vi "VNA-FMR-POLREF_(LV2017).vi"() -> ()   [LabVIEW 2017] (continued)
  out "XY Graph 3":cluster{"Trace Data":dbl[], "Trace Data":dbl[]}(graph)
  in  "RF State (T) 2":bool=TRUE caption="RF State (T)"
  in  "Bandwidth":dbl=400.0 caption="Bandwidth (10.0e3)" format="%#.9p"
  in  "Sweep Time":dbl=8.0 caption="Sweep Time (21.909e-3)" format="%^.3e"
  in  "Auto Sweep Time":bool caption="Auto Sweep Time (T)"
  in  "Power":dbl=-2.0 caption="Power (-10.0)" format="%^.3e"
  in  "Number Of Points":i32=1601
  in  "Display 2":bool=TRUE
  out "Current value":dbl=0.2540000081062317
  out "Range 4":dbl
  out "Units 6":dbl
  out "Mode 4":dbl=1.0
  in  "Commit 2":bool caption="Commit"
  out "Formatted value":dbl=0.2540000081062317 format="%3_4p"
  out "Units 5":string="T"
  in  "Range 3":i32(knob) scale=0.0..4.0
  in  "Mode 3":u32(knob) scale=0.0..4.0
  in  "Units 4":u32(knob) scale=0.0..3.0
  out "Ba Stability":string="wait"
  out "Actual Current Level (A)":dbl=8.81 format="%.2g"
  out "output matrix 2":T1
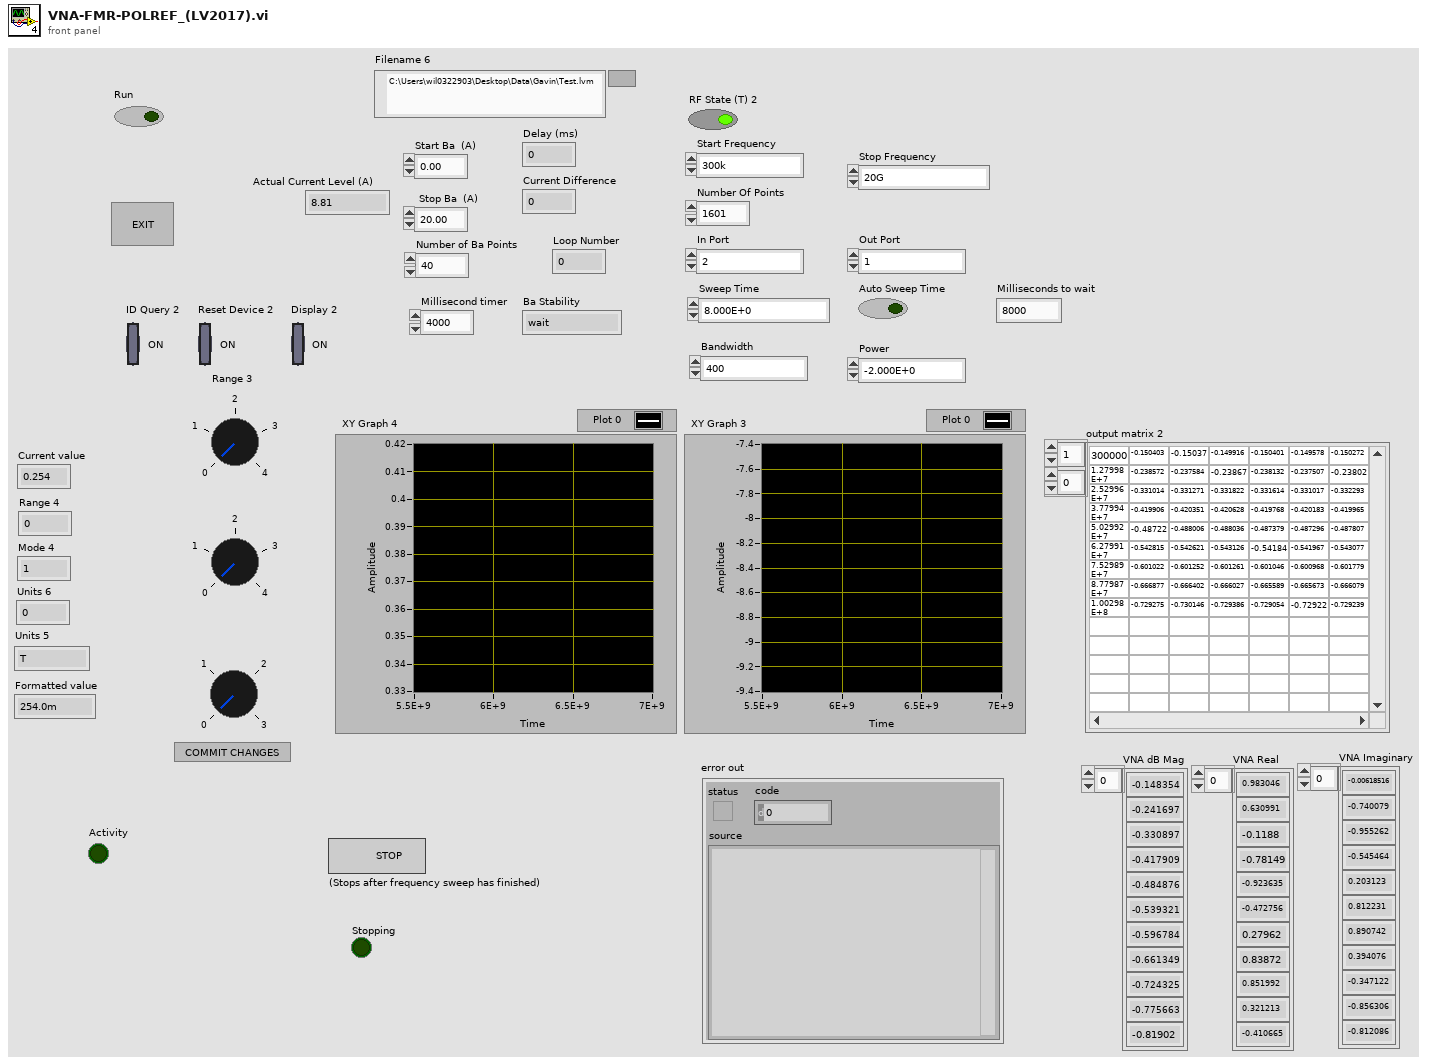
[diagram p1: front panel]
types:
  T1 = typedef "NI_Matrix.lvlib/RealMatrix.ctl" = dbl[][]
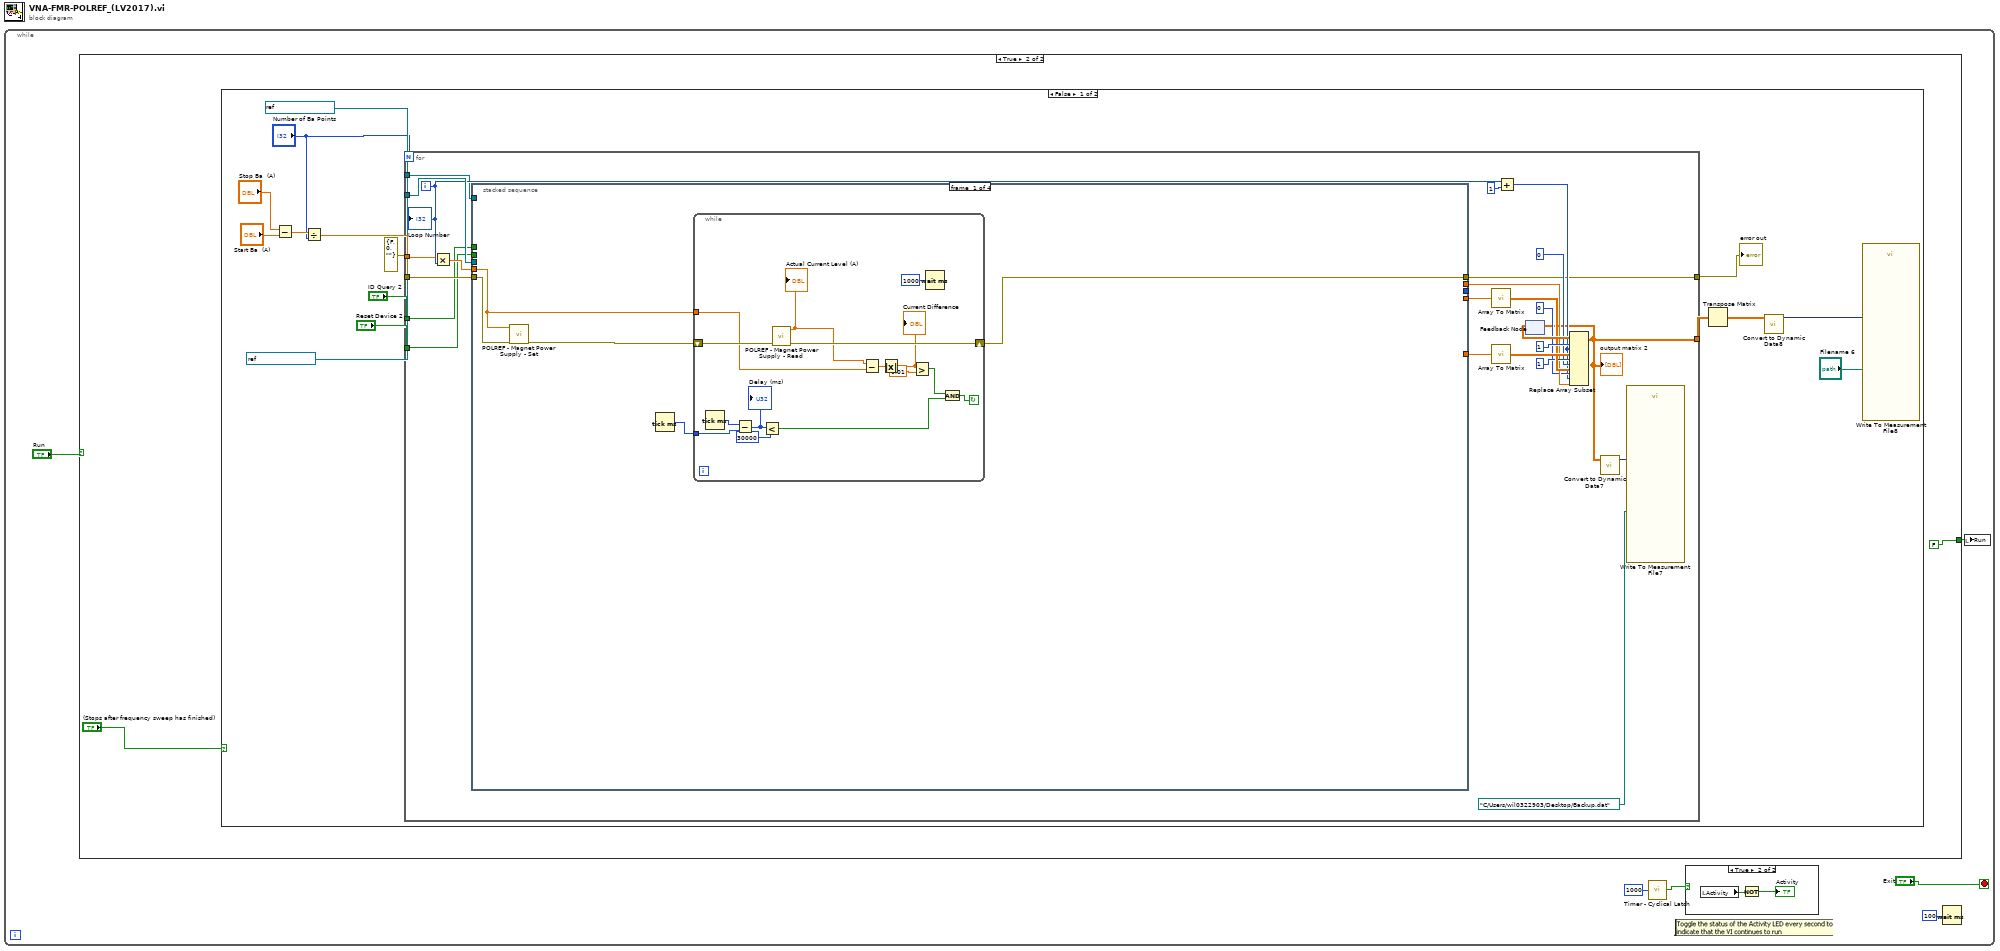
[diagram p0: block diagram]
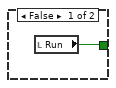
[diagram p3: hidden frame]
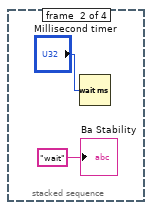
[diagram p4: hidden frame]
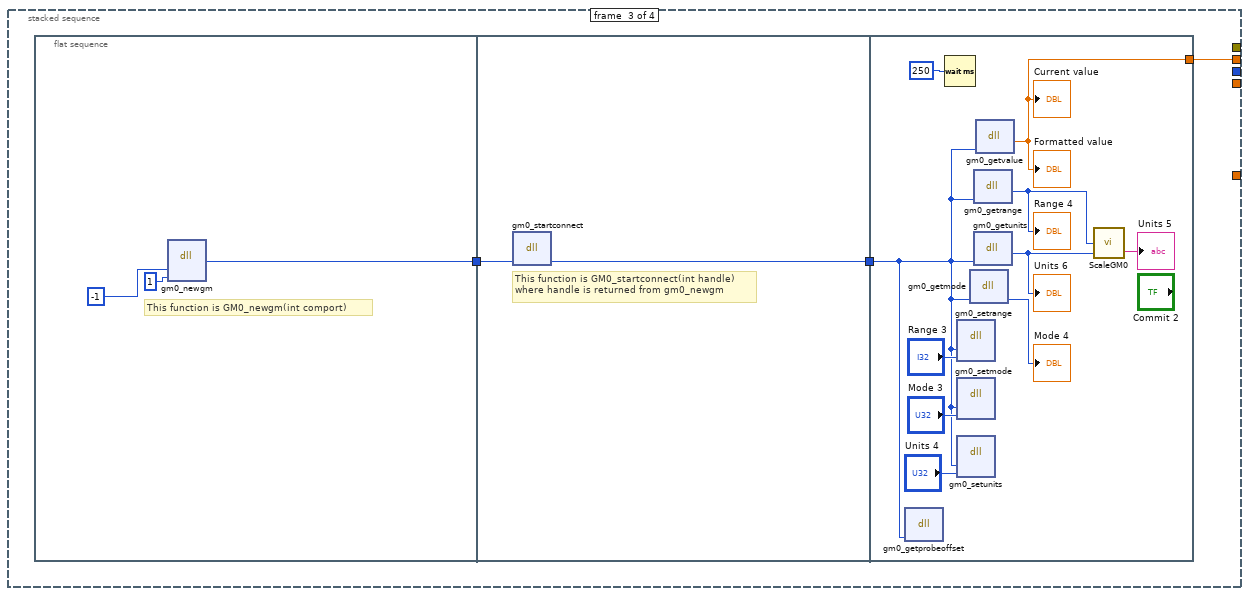
[diagram p5: hidden frame]
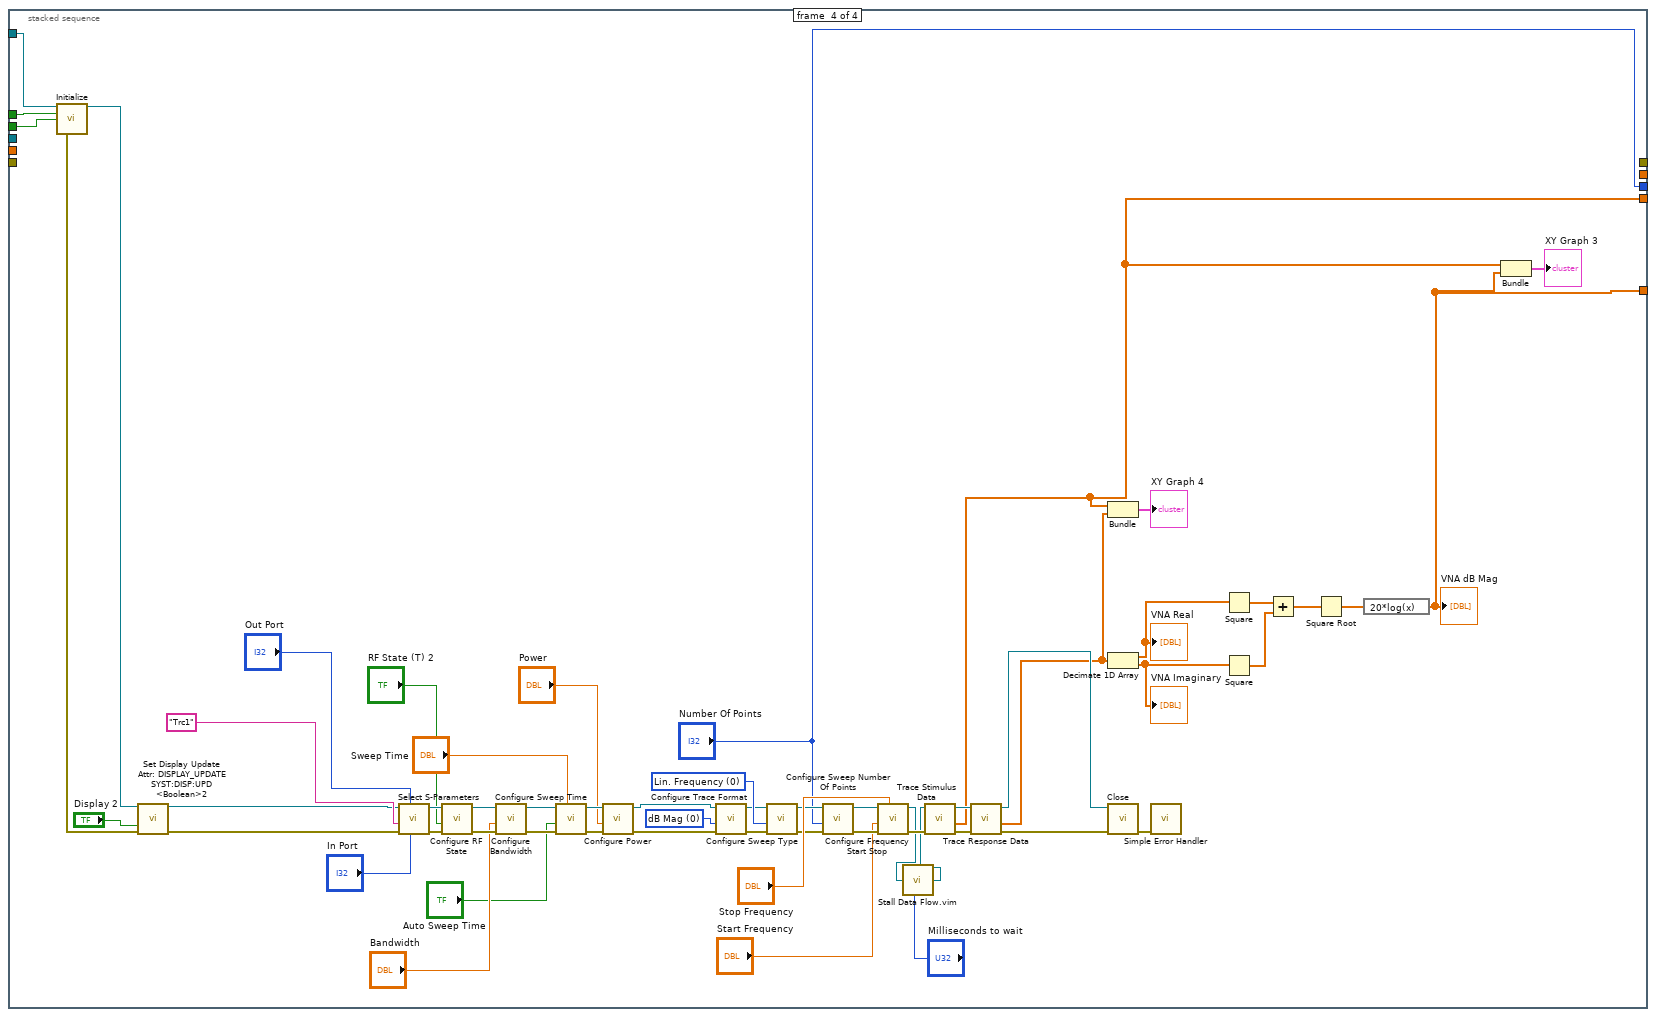
[diagram p6: hidden frame]
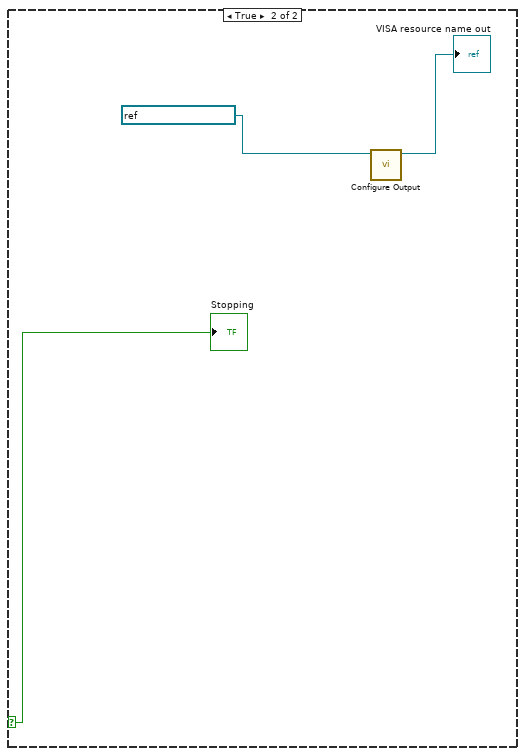
[diagram p7: hidden frame]
diagram:
  n1 = while {
    stop <- "Exit" stop-if-true
    n2 = case shown="True" "Run" {
      tunnel: [w9 FALSE ("Run Button")] -> w1
      frame False {
        n3 = local read "Run"() -> (w9:bool)
      }
      frame True {
        n4 = case shown="False" "(Stops after frequency sweep has finished)" {
          selector: "(Stops after frequency sweep has finished)" -> [_ w150]
          frame False {
            n5 = Subtract(x="Stop Ba  (A)", y="Start Ba  (A)") -> (x-y=w18:dbl)
            n6 = Divide(x=w18, y="Number of Ba Points") -> (x/y=w16:dbl)
            n7 = for {
              N: "Number of Ba Points" -> [_]
              tunnel: [w36] -> w24
              tunnel: w16 -> [w32]
              tunnel: errorcluster {"status"=FALSE, "code"=0, "source"=""} ("error in (no error)") -> [w35]
              tunnel: refnum<visa-resource-name> "GPIB1::11::INSTR" ("VISA resource name 3") -> [w34]
              tunnel: refnum<visa-resource-name> "GPIB1::20::INSTR" ("VISA resource name 2") -> [w30]
              tunnel: "ID Query 2" -> [w29]
              tunnel: "Reset Device 2" -> [w28]
              tunnel: [w27] -> w12
              i -> [w33]
              n8 = Multiply(x=w32, y=w33) -> (x*y=w31:dbl)
              n9 = stacked-sequence {
                tunnel: [_ _ w73 _] -> w41
                tunnel: [_ _ _ w104] -> w49
                tunnel: [_ _ _ w103] -> w50
                tunnel: [_ _ _ "Number Of Points"] -> _
                tunnel: w34 -> [_ _ _ _]
                tunnel: w35 -> [w55 _ _ _]
                tunnel: w31 -> [w52 _ _ _]
                tunnel: w30 -> [_ _ _ w99]
                tunnel: w29 -> [_ _ _ w98]
                tunnel: w28 -> [_ _ _ w97]
                tunnel: [w53 _ _ _] -> w27
                frame #0 {
                  n10 = call "POLREF - Magnet Power Supply - Set.vi"("error in (no error)"=w55, "Magnet Current - Set"=w52) -> ("error out"=w54:errorcluster)  [unwired: 9 in]
                  n11 = Tick Count (ms)() -> (millisecond timer value=w51:u32)
                  n12 = while {
                    shift-right: [w69] -> w53
                    shift-left: w54 -> [w70]
                    tunnel: w52 -> [w67]
                    tunnel: w51 -> [w61]
                    stop <- w57 continue-if-true
                    n13 = Tick Count (ms)() -> (millisecond timer value=w62:u32)
                    n14 = Subtract(x=w62, y=w61) -> (x-y=w60:u32)
                    "Delay (ms)" <- w60
                    n15 = Less?(x=w60, y=u32 30000) -> (x < y?=w58:bool)
                    n16 = call "POLREF - Magnet Power Supply - Read.vi"("error in (no error)"=w70) -> ("error out"=w69:errorcluster, "Magnet Current"=w68:dbl)  [unwired: 9 in]
                    "Actual Current Level (A)" <- w68
                    n17 = Subtract(x=w68, y=w67) -> (x-y=w66:dbl)
                    n18 = Absolute Value(x=w66) -> (abs(x)=w65:dbl)
                    "Current Difference" <- w65
                    n19 = Greater?(x=w65, y=0.01) -> (0:w56:bool)
                    n20 = Wait (ms)(milliseconds to wait=u32 1000) -> ()  [unwired: 1 out]
                    n21 = Compound Arithmetic op=AND(w56, w58) -> (w57:bool)
                  }
                }
                frame #1 {
                  n22 = Wait (ms)(milliseconds to wait="Millisecond timer") -> ()  [unwired: 1 out]
                  "Ba Stability" <- "wait"
                }
                frame #2 {
                  n23 = flat-sequence {
                    tunnel: [w76] -> w75
                    tunnel: w75 -> [w79]
                    tunnel: [w80] -> w74
                    tunnel: w74 -> [w82]
                    tunnel: [w81] -> w73
                    frame #0 {
                      # "This function is GM0_newgm(int comport)"
                      n24 = dll-call lib="C:/Users/wil0322903/Desktop/Hall Probe/LabView-VI/gm0.dll" fn="gm0_newgm"("comport"=-1 ("Com Port 2"), "mode"=1) -> ("handle"=w76:i32)  [unwired: 5 in, 2 out]
                    }
                    frame #1 {
                      # "This function is GM0_startconnect(int handle)\nwhere handle is returned from gm0_newgm"
                      n25 = dll-call lib="C:/Users/wil0322903/Desktop/Hall Probe/LabView-VI/gm0.dll" fn="gm0_startconnect"("handle"=w79) -> ("handle"=w80:i32)  [unwired: 4 in, 2 out]
                    }
                    frame #2 {
                      n26 = dll-call lib="C:/Users/wil0322903/Desktop/Hall Probe/LabView-VI/gm0.dll" fn="gm0_getprobeoffset"("handle"=w82) -> ()  [unwired: 5 in, 2 out]
                      n27 = Wait (ms)(milliseconds to wait=250) -> ()  [unwired: 1 out]
                      n28 = dll-call lib="C:/Users/wil0322903/Desktop/Hall Probe/LabView-VI/gm0.dll" fn="gm0_setrange"("handle"=w82, "new range"="Range 3") -> ()  [unwired: 6 in, 2 out]
                      n29 = dll-call lib="C:/Users/wil0322903/Desktop/Hall Probe/LabView-VI/gm0.dll" fn="gm0_setmode"("handle"=w82, "new mode"="Mode 3") -> ()  [unwired: 6 in, 2 out]
                      n30 = dll-call lib="C:/Users/wil0322903/Desktop/Hall Probe/LabView-VI/gm0.dll" fn="gm0_setunits"("handle"=w82, "new units"="Units 4") -> ()  [unwired: 6 in, 2 out]
                      n31 = dll-call lib="C:/Users/wil0322903/Desktop/Hall Probe/LabView-VI/gm0.dll" fn="gm0_getmode"("handle"=w82) -> ("handle"=→"Mode 4":i32)  [unwired: 4 in, 2 out]
                      n32 = dll-call lib="C:/Users/wil0322903/Desktop/Hall Probe/LabView-VI/gm0.dll" fn="gm0_getrange"("handle"=w82) -> ("value"=w88:i32)  [unwired: 4 in, 2 out]
                      "Range 4" <- w88
                      n33 = dll-call lib="C:/Users/wil0322903/Desktop/Hall Probe/LabView-VI/gm0.dll" fn="gm0_getunits"("handle"=w82) -> ("units"=w87:i32)  [unwired: 4 in, 2 out]
                      "Units 6" <- w87
                      n34 = dll-call lib="C:/Users/wil0322903/Desktop/Hall Probe/LabView-VI/gm0.dll" fn="gm0_getvalue"("handle"=w82) -> ("value"=w81:dbl)  [unwired: 4 in, 2 out]
                      "Current value" <- w81
                      "Formatted value" <- w81
                      n35 = call "ScaleGM0.vi"("Units"=w87, "Range"=w88) -> ("Units"=→"Units 5":string)  [unwired: 1 in, 1 out]
                    }
                  }
                }
                frame #3 {
                  w141 = 0 items=["Lin. Frequency", "Log. Frequency", "Segmented Frequency", "Power", "Time", "CW Mode"] ("Sweep Type (Power)")
                  w142 = 0 items=["dB Mag", "Phase", "Smith", "Polar", "Delay", "SWR", "Lin Mag", "Real", "Imag", "Inverted Smith", "Unwrapped Phase"] ("Format (dB Mag)")
                  n36 = call <instrlib>:"Initialize.vi"("VISA resource name"=w99, "ID Query (T: Check)"=w98, "Reset (T: Reset)"=w97) -> ("VISA resource name out"=w94:refnum<visa-resource-name>, "error out"=w101:errorcluster)  [unwired: 11 in]
                  n37 = call "Set Display Update \nAttr: DISPLAY_UPDATE\nSYST:DISP:UPD <Boolean>2"("instrument handle"=w94, "Display Update (OFF)"="Display 2", "error in (no error)"=w101) -> ("instrument handle out"=w96:refnum<visa-resource-name>, "error out"=w95:errorcluster)  [unwired: 11 in]
                  n38 = call <instrlib>:"Select S-Parameters.vi"("In Port (1)"="In Port", "Out Port (1)"="Out Port", "error in (no error)"=w95, "Trace Name (\"Trc1\")"="Trc1" ("Trace Name (\"Trc1\") 2"), "VISA resource name"=w96) -> ("error out"=w116:errorcluster, "VISA resource name out"=w119:refnum<visa-resource-name>)  [unwired: 5 in]
                  n39 = call <instrlib>:"Configure RF State.vi"("error in (no error)"=w116, "RF State (T)"="RF State (T) 2", "VISA resource name"=w119) -> ("error out"=w115:errorcluster, "VISA resource name out"=w118:refnum<visa-resource-name>)  [unwired: 7 in]
                  n40 = call <instrlib>:"Configure Bandwidth.vi"("error in (no error)"=w115, "Bandwidth (10kHz)"="Bandwidth", "VISA resource name"=w118) -> ("error out"=w114:errorcluster, "VISA resource name out"=w117:refnum<visa-resource-name>)  [unwired: 7 in]
                  n41 = call <instrlib>:"Configure Sweep Time.vi"("Sweep Time (21.909e-3)"="Sweep Time", "error in (no error)"=w114, "Auto Sweep Time (T)"="Auto Sweep Time", "VISA resource name"=w117) -> ("error out"=w108:errorcluster, "VISA resource name out"=w109:refnum<visa-resource-name>)  [unwired: 6 in]
                  n42 = call <instrlib>:"Configure Power.vi"("error in (no error)"=w108, "Power (-10.0)"="Power", "VISA resource name"=w109) -> ("error out"=w106:errorcluster, "VISA resource name out"=w107:refnum<visa-resource-name>)  [unwired: 7 in]
                  n43 = call <instrlib>:"Configure Trace Format.vi"("error in (no error)"=w106, "Format (dB Mag)"=w142, "VISA resource name"=w107) -> ("error out"=w138:errorcluster, "VISA resource name out"=w140:refnum<visa-resource-name>)  [unwired: 7 in]
                  n44 = call <instrlib>:"Configure Sweep Type.vi"("error in (no error)"=w138, "Sweep Type (Power)"=w141, "VISA resource name"=w140) -> ("error out"=w137:errorcluster, "VISA resource name out"=w139:refnum<visa-resource-name>)  [unwired: 7 in]
                  n45 = call <instrlib>:"Configure Sweep Number Of Points.vi"("error in (no error)"=w137, "Number Of Points (201)"="Number Of Points", "VISA resource name"=w139) -> ("error out"=w145:errorcluster, "VISA resource name out"=w146:refnum<visa-resource-name>)  [unwired: 7 in]
                  n46 = call <instrlib>:"Configure Frequency Start Stop.vi"("Stop Frequency (4GHz)"="Stop Frequency", "error in (no error)"=w145, "Start Frequency (300kHz)"="Start Frequency", "VISA resource name"=w146) -> ("error out"=w133:errorcluster, "VISA resource name out"=w92:refnum<visa-resource-name>)  [unwired: 6 in]
                  n47 = call "Stall Data Flow.vim"("value in"=w92, "milliseconds to wait"="Milliseconds to wait") -> ("value out"=w91:refnum<visa-resource-name>)  [unwired: 1 out]
                  n48 = call <instrlib>:"Trace Stimulus Data.vi"("error in (no error)"=w133, "VISA resource name"=w91) -> ("error out"=w128:errorcluster, "Trace Data"=w103:dbl[], "VISA resource name out"=w131:refnum<visa-resource-name>)  [unwired: 6 in, 1 out]
                  n49 = call <instrlib>:"Trace Response Data.vi"("error in (no error)"=w128, "VISA resource name"=w131) -> ("error out"=w129:errorcluster, "Trace Data"=w127:dbl[], "VISA resource name out"=w130:refnum<visa-resource-name>)  [unwired: 6 in, 1 out]
                  n50 = Bundle("Trace Data"=w103, "Trace Data"=w127) -> (→"XY Graph 4":cluster{"Trace Data":dbl[], "Trace Data":dbl[]})  [unwired: 1 in]
                  n51 = Decimate 1D Array(w127) -> (w125:dbl[], w126:dbl[])
                  "VNA Real" <- w125
                  "VNA Imaginary" <- w126
                  n52 = call <instrlib>:"Close.vi"("error in (no error)"=w129, "VISA resource name"=w130) -> ("error out"=w147:errorcluster)  [unwired: 9 in]
                  n53 = call <vilib>:"Simple Error Handler.vi"("error in (no error)"=w147) -> ()  [unwired: 4 in, 5 out]
                  n54 = Square(x=w125) -> (x^2=w123:dbl[])
                  n55 = Square(x=w126) -> (x^2=w124:dbl[])
                  n56 = Add(x=w123, y=w124) -> (x+y=w122:dbl[])
                  n57 = Square Root(x=w122) -> (sqrt(x)=w121:dbl[])
                  n58 = expression code="20*log(x)"(w121) -> (w104:dbl[])
                  "VNA dB Mag" <- w104
                  n59 = Bundle("Trace Data"=w103, w104) -> (→"XY Graph 3":cluster{"Trace Data":dbl[], dbl[]})  [unwired: 1 in]
                }
              }
              n60 = call-poly <vilib>:"Array To Matrix.vi"("Real 1D Array"=w50) -> ("Real Matrix (Column Vector)"=w44:T1)
              n61 = call-poly <vilib>:"Array To Matrix.vi"("Real 1D Array"=w49) -> ("Real Matrix (Column Vector)"=w46:T1)
              n62 = Add(x=w33, y=1) -> (x+y=w39:i32)
              n63 = feedback #1() -> (w45:T1)  [unwired: 1 in]
              n64 = Replace Array Subset(array=w45, new element #1=w46, index (row) #1=1 ("disabled index (row)"), index (col) #1=w39, new element #2=w44, index (row) #2=1 ("index (row)"), index (col) #2=0 ("disabled index (col)"), new element #3=w41, index (row) #3=0 ("index (row)"), index (col) #3=w39) -> (w36:T1)
              "output matrix 2" <- w36
              n65 = feedback-in #1(w36) -> ()
              n66 = call "Convert to Dynamic Data7"("2D Array"=w36) -> ("Dynamic Data Type"=w38:dynamicdata)  [unwired: 3 in]
              n67 = call "Write To Measurement File7"("Signals"=w38, "Filename"=path "C:/Users/wil0322903/Desktop/Backup.dat" ("Filename 4")) -> ()  [unwired: 15 in, 3 out]
              "Loop Number" <- w33
            }
            "error out" <- w12
            n68 = Transpose Matrix(1:w24) -> (0:w23:T1)
            n69 = call "Convert to Dynamic Data8"("2D Array"=w23) -> ("Dynamic Data Type"=w26:dynamicdata)  [unwired: 3 in]
            n70 = call "Write To Measurement File8"("Signals"=w26, "Filename"="Filename 6") -> ()  [unwired: 15 in, 3 out]
          }
          frame True {
            n71 = call <instrlib>:"Configure Output.vi"("VISA resource name"=refnum<visa-resource-name> "GPIB0::11::INSTR" ("VISA resource name 2")) -> ("VISA resource name out"=→"VISA resource name out":refnum<visa-resource-name>)  [unwired: 9 in, 1 out]
            "Stopping" <- w150
          }
        }
      }
    }
    n72 = call "Timer - Cyclical Latch.vi"("Timer (msec)"=u32 1000) -> ("Timer Trigger"=w3:bool)  [unwired: 14 in]
    n73 = case shown="True" w3 {
      frame False {
      }
      frame True {
        n74 = local read "Activity"() -> (w7:bool)
        n75 = Not(x=w7) -> (.not. x?=→"Activity":bool)
      }
    }
    n76 = Wait (ms)(milliseconds to wait=u32 100) -> ()  [unwired: 1 out]
    n77 = local write "Run"(w1) -> ()
  }
